vi "UHR-Fleezers Control (host) - 12.7b.vi"() -> ()   [LabVIEW 2012] (continued)
        n815 = case shown="True" w1258 {
          tunnel: w1261 -> [_ w1264]
          tunnel: "Fish for Tether" -> [_ w1263]
          frame False {
          }
          frame True {
            n816 = case shown="True" w1263 {
              selector: w1263 -> [w1267 w1273]
              tunnel: [w1267 w1273] -> w1262
              frame False {
              }
              frame True {
                n817 = local write "Scan axis 2"(TRUE) -> ()
                n818 = local write "Tether"(FALSE ("Tether")) -> ()
                n819 = local read "Flow ON during cal?"() -> (w1268:bool)
                n820 = property on="Trap Delta (MHz)" class="DigNum (strict)"("Val(Sgnl)"="Furthest Delta (MHz)") -> ()  [unwired: 2 in, 2 out]
                n821 = Or(x="Flow ON during \nfishing?", y=w1268) -> (x .or. y?=w1269:bool)
                n822 = Wait (ms)(milliseconds to wait=u32 500) -> ()  [unwired: 1 out]
                n823 = property on="Sample Channel\nFlow" class="Bool (strict)"("Val(Sgnl)"=w1269) -> ()  [unwired: 2 in, 2 out]
              }
            }
            n824 = node-c288() -> (w1266:T23)  [unwired: 1 in, 3 out]
            n825 = timed-loop "Oscillate AOD" {
              timing: w1266 -> [_]
              timing-out: [_] -> w1265
              tunnel: w1264 -> [w1283]
              tunnel: w1262 -> [w1276]
              i -> [w1285]
              stop <- w1282 stop-if-true
              n826 = node-c288() -> (w1284:i64)  [unwired: 1 out]
              n827 = flat-sequence {
                tunnel: w1285 -> [w1312]
                tunnel: w1284 -> [w1311]
                tunnel: w1283 -> [w1293]
                tunnel: w1276 -> [w1295]
                tunnel: [w1295] -> w1281
                tunnel: [w1294] -> w1280
                tunnel: [w1292] -> w1279
                tunnel: [w1289] -> w1277
                tunnel: w1281 -> [w1357]
                tunnel: w1280 -> [w1355]
                tunnel: w1279 -> [w1354]
                tunnel: [w1353] -> w1278
                tunnel: w1277 -> [w1352]
                tunnel: [w1429] -> w1282
                tunnel: w1278 -> [w1428]
                frame #0 {
                  # "w (rad/s)"
                  # "t (s)"
                  n828 = Divide(x=w1311, y=i64 1000) -> (x/y=w1286:dbl)
                  n829 = local read "BD 1 Frequency 2 (MHz)"() -> (w1288:dbl)
                  n830 = Multiply(x="Osc. freq. (Hz)", y=6.283185307179586) -> (x*y=w1309:dbl)
                  n831 = Multiply(x=w1286, y=w1312) -> (x*y=w1308:dbl)
                  n832 = Multiply(x=w1309, y=w1308) -> (x*y=w1291:dbl)
                  n833 = local read "BD 1 Frequency 1 (MHz)"() -> (w1297:dbl)
                  n834 = case shown="True" w1295 {
                    tunnel: w1291 -> [w1318 w1335]
                    tunnel: w1297 -> [_ w1343]
                    tunnel: w1288 -> [_ w1344]
                    tunnel: [w1315 w1339] -> w1287
                    tunnel: [FALSE w1320] -> w1292
                    tunnel: [0.0 w1331] -> w1289
                    frame False {
                      n835 = Sine(x=w1318) -> (sin(x)=w1316:dbl)
                      n836 = Multiply(x=w1316, y="Osc. amp. (MHz)") -> (x*y=w1315:dbl)
                    }
                    frame True {
                      # "trap position goes from 0 to 1 (0 is when it is furthest away, 1 is when closest)\nso we want to test for tether only when farther away, or x < 1"
                      # "quit if taking too long"
                      # "oscillate the trap"
                      # "Test for tether"
                      n837 = local read "Vec Mean of T1 T2"() -> (w1319:dbl[])
                      "Trigger Signal" <- w1319
                      n838 = Cosine(x=w1335) -> (cos(x)=w1347:dbl)
                      n839 = Subtract(x=w1344, y=w1343) -> (x-y=w1342:dbl)
                      n840 = Decrement(x=w1347) -> (x-1=w1346:dbl)
                      n841 = Subtract(x=w1342, y="Closest Delta (MHz)") -> (x-y=w1340:dbl)
                      n842 = Divide(x=w1346, y=-2.0) -> (x/y=w1330:dbl)
                      n843 = Greater?(x=w1319, y="Stop F (pN)") -> (0:w1337:bool[])
                      n844 = Multiply(x=w1330, y=w1340) -> (x*y=w1339:dbl)
                      n845 = Less?(x=w1330, y="Fish mask thresh") -> (x < y?=w1329:bool)
                      n846 = Boolean To (0,1)(Boolean=w1329) -> (0, 1=w1327:i16)
                      n847 = Multiply(x=w1327, y=w1319) -> (x*y=w1326:dbl[])
                      n848 = Divide(x=w1335, y=6.283185307179586) -> (x/y=w1334:dbl)
                      n849 = Round Toward +Infinity(x=w1334) -> (ceil(x): smallest int >= x=w1331:dbl)
                      "Attempts" <- w1331
                      n850 = Greater?(x=w1326, y="Stop F (pN) (mask)") -> (0:w1324:bool[])
                      n851 = Or Array Elements(Boolean array=w1337) -> (logical OR=w1322:bool)
                      n852 = Or Array Elements(Boolean array=w1324) -> (logical OR=w1321:bool)
                      n853 = Greater?(x=w1331, y="Attempt Limit") -> (0:w1333:bool)
                      n854 = case shown="True" w1333 {
                        frame False {
                        }
                        frame True {
                          n855 = local write "Fish for Tether"(FALSE ("Fish for Tether")) -> ()
                          n856 = call <vilib>:"Beep.vi"() -> ()  [unwired: 3 in, 9 out]
                          n857 = local read "Messages"() -> (w1349:string)
                          n858 = call "Update messages.vi"("Message to add"="Tether fishing timeout." ("Messages"), "Old message string"=w1349) -> ("New message string"=→"Messages":string)
                        }
                      }
                      n859 = Select(t=w1322, s="Normal (on) or masked test (off)", f=w1321) -> (s? t:f=w1320:bool)
                    }
                  }
                  n860 = local read "BD 2 Frequency 1 (MHz)"() -> (w1296:dbl)
                  n861 = Select(t=w1297, s="Scan axis 2", f=w1296) -> (s? t:f=w1300:dbl)
                  n862 = Add(x=w1287, y=w1300) -> (x+y=w1294:dbl)
                  n863 = Select(t=w1294, s="Scan axis 2", f=w1297) -> (s? t:f=w1303:dbl)
                  n864 = Select(t=w1296, s="Scan axis 2", f=w1294) -> (s? t:f=w1302:dbl)
                  n865 = local read "BD 2 Frequency 2 (MHz)"() -> (w1305:dbl)
                  n866 = local read "BD 2 Frequency 3 (MHz)"() -> (w1304:dbl)
                  n867 = local read "Y RF Frequency Limits (MHz)"() -> (w1298:T16)
                  n868 = local read "X RF Frequency Limits (MHz)"() -> (w1299:T16)
                  n869 = local read "BD 1 Frequency 3 (MHz)"() -> (w1306:dbl)
                  n870 = call "set RF board frequency - interlace.vi"("Board 2 Frequency Limits"=w1298, "Board 1 Frequency Limits"=w1299, "FPGA VI Reference In"=w1293, "Board 2 Frequency 3 (MHz)"=w1304, "Board 1 Frequency 3 (MHz)"=w1306, "Board 2 Frequency 2 (MHz)"=w1305, "Board 2 Frequency 1 (MHz)"=w1302, "Board 1 Frequency 2 (MHz)"=w1288, "Board 1 Frequency 1  (MHz)"=w1303) -> ()  [unwired: 1 in, 2 out]
                }
                frame #1 {
                  n871 = And(x=w1357, y=w1354) -> (x .and. y?=w1356:bool)
                  n872 = case "Only if were fishing and now formed tether" shown="True" w1356 {
                    tunnel: w1355 -> [w1359 w1374]
                    tunnel: [w1358 w1373] -> w1353
                    tunnel: w1352 -> [_ w1369]
                    frame False {
                      n873 = local read "Fish for Tether"() -> (w1358:bool)
                      n874 = case shown="False" w1358 {
                        tunnel: w1359 -> [w1360 _]
                        frame False {
                          n875 = property on="BD 1 Frequency 1 (MHz)" class="DigNum (strict)"("Val(Sgnl)"=w1360) -> ()  [unwired: 2 in, 2 out]
                        }
                        frame True {
                        }
                      }
                    }
                    frame True {
                      w1373 = FALSE ("Fish for Tether")
                      n876 = call <vilib>:"Beep.vi"() -> ()  [unwired: 3 in, 9 out]
                      n877 = Number To Decimal String(number=w1369, width (-)=i16 1) -> (decimal integer string=w1367:string)
                      n878 = Concatenate Strings("Formed tether in ", w1367, " attempt(s)." ("string")) -> (w1364:string)
                      n879 = local read "Messages"() -> (w1371:string)
                      n880 = local write "Fish for Tether"(w1373) -> ()
                      n881 = call "Update messages.vi"("Message to add"=w1364, "Old message string"=w1371) -> ("New message string"=w1370:string)
                      n882 = local write "Messages"(w1370) -> ()
                      n883 = Get Date/Time In Seconds() -> (seconds since 1Jan1904=→"Time tether formed":timestamp)
                      n884 = local read "Flow ON during cal?"() -> (w1361:bool)
                      n885 = property on="Sample Channel\nFlow" class="Bool (strict)"("Val(Sgnl)"=w1361) -> (error out=w1362:errorcluster)  [unwired: 2 in, 1 out]
                      n886 = case shown="\"2\", \"3\", \"4\", \"5\", \"6\"" "Then..." {
                        selector: "Then..." -> [_ w1377]
                        tunnel: w1374 -> [w1376 _]
                        tunnel: w1362 -> [_ _]
                        frame "1", Default {
                          n887 = property on="BD 1 Frequency 1 (MHz)" class="DigNum (strict)"("Val(Sgnl)"=w1376) -> ()  [unwired: 2 in, 2 out]
                        }
                        frame "2", "3", "4", "5", "6" {
                          n888 = flat-sequence {
                            tunnel: w1377 -> [w1379]
                            frame #0 {
                              n889 = property on="Trap Delta (MHz)" class="DigNum (strict)"("Val(Sgnl)"="Move to Delta 1 (MHz)") -> ()  [unwired: 2 in, 2 out]
                            }
                            frame #1 {
                              n890 = case shown="\"5\", \"6\"" w1379 {
                                selector: w1379 -> [w1382 w1392 _]
                                frame "3", "4" {
                                n891 = flat-sequence {
                                tunnel: w1382 -> [w1383]
                                tunnel: [w1383] -> w1380
                                tunnel: [w1385] -> w1381
                                tunnel: w1380 -> [w1385]
                                tunnel: w1381 -> [w1389]
                                frame #0 {
                                n892 = property on="Green Laser ON" class="Bool (strict)"("Val(Sgnl)"=TRUE ("Value (Signaling)")) -> ()  [unwired: 2 in, 2 out]
                                }
                                frame #1 {
                                n893 = Multiply(x="Wait Before Save (s)", y=u32 1000 ("x")) -> (x*y=w1387:u32)
                                n894 = Wait (ms)(milliseconds to wait=w1387) -> ()  [unwired: 1 out]
                                }
                                frame #2 {
                                n895 = property on="Start Saving" class="Bool (strict)"("Value"=TRUE ("Start Saving")) -> ()  [unwired: 2 in, 2 out]
                                n896 = case shown="\"4\"" w1389 {
                                frame Default {
                                }
                                frame "4" {
                                n897 = property on="Fl. Triggered..." class="Bool (strict)"("Val(Sgnl)"=TRUE ("Value (Signaling)")) -> ()  [unwired: 2 in, 2 out]
                                }
                                }
                                }
                                }
                                }
                                frame "5", "6" {
                                n898 = stacked-sequence {
                                tunnel: w1392 -> [_ _ _ _ _ _ w1404]
                                frame #0 {
                                n899 = Replace Array Subset(array=u32[] [0] ("Index Values"), new element="Raster Set Upon Tether", index=0) -> (w1393:u32[])
                                n900 = property on="Saved AOD Raster Scan Parameter Sets" class="Arr (strict)"("Index Values"=w1393) -> ()  [unwired: 2 in, 2 out]
                                }
                                frame #1 {
                                n901 = Wait (ms)(milliseconds to wait=u32 500) -> ()  [unwired: 1 out]
                                }
                                frame #2 {
                                n902 = property on="Load parameters" class="Bool (strict)"("Val(Sgnl)"=TRUE ("Value (Signaling)")) -> ()  [unwired: 2 in, 2 out]
                                n903 = case shown="True" "Green ON During Raster" {
                                frame False {
                                }
                                frame True {
                                n904 = property on="Green Laser ON" class="Bool (strict)"("Val(Sgnl)"=TRUE ("Value (Signaling)")) -> ()  [unwired: 2 in, 2 out]
                                }
                                }
                                }
                                frame #3 {
                                n905 = Wait (ms)(milliseconds to wait=u32 500) -> ()  [unwired: 1 out]
                                }
                                frame #4 {
                                n906 = property on="Trap Raster Scan" class="Bool (strict)"("Val(Sgnl)"=TRUE ("Value (Signaling)")) -> ()  [unwired: 2 in, 2 out]
                                }
                                frame #5 {
                                n907 = Wait (ms)(milliseconds to wait=u32 2000) -> ()  [unwired: 1 out]
                                }
                                frame #6 {
                                n908 = flat-sequence {
                                tunnel: w1404 -> [w1411]
                                frame #0 {
                                n909 = while {
                                stop <- w1407 stop-if-true
                                n910 = local read "Raster Scanning..."() -> (w1406:bool)
                                n911 = local read "Saving..."() -> (w1409:bool)
                                n912 = Wait (ms)(milliseconds to wait=u32 100) -> ()  [unwired: 1 out]
                                n913 = Not(x=w1409) -> (.not. x?=w1408:bool)
                                n914 = Not(x=w1406) -> (.not. x?=w1405:bool)
                                n915 = And(x=w1408, y=w1405) -> (x .and. y?=w1407:bool)
                                }
                                }
                                frame #1 {
                                n916 = local read "Tether"() -> (w1412:bool)
                                n917 = case shown="True" w1412 {
                                tunnel: w1411 -> [_ w1414]
                                frame False {
                                n918 = property on="Fish for Tether" class="Bool (strict)"("Val(Sgnl)"="Fish again after \nraster break?") -> ()  [unwired: 2 in, 2 out]
                                }
                                frame True {
                                n919 = stacked-sequence {
                                tunnel: w1414 -> [_ w1418 _ _]
                                frame #0 {
                                n920 = property on="Trap Delta (MHz)" class="DigNum (strict)"("Val(Sgnl)"="Move to Delta 2 (MHz)") -> ()  [unwired: 2 in, 2 out]
                                n921 = case shown="True" "Flow ON after\ntether testing?" {
                                frame False {
                                }
                                frame True {
                                n922 = property on="Sample Channel\nFlow" class="Bool (strict)"("Val(Sgnl)"=TRUE ("Value (Signaling)")) -> ()  [unwired: 2 in, 2 out]
                                }
                                }
                                }
                                frame #1 {
                                n923 = flat-sequence {
                                tunnel: w1418 -> [w1420]
                                frame #0 {
                                n924 = Wait (ms)(milliseconds to wait=u32 500) -> ()  [unwired: 1 out]
                                }
                                frame #1 {
                                n925 = case shown="\"6\"" w1420 {
                                frame Default {
                                }
                                frame "6" {
                                n926 = property on="Green Laser ON" class="Bool (strict)"("Val(Sgnl)"=TRUE ("Green Laser ON/Interlacing")) -> ()  [unwired: 2 in, 2 out]
                                }
                                }
                                }
                                frame #2 {
                                n927 = Wait (ms)(milliseconds to wait=u32 500) -> ()  [unwired: 1 out]
                                }
                                frame #3 {
                                n928 = local write "Start Saving"("Save at end (5, 6)") -> ()
                                }
                                }
                                }
                                frame #2 {
                                n929 = local read "Bead Sep. Int. Time (s)"() -> (w1426:dbl)
                                n930 = Multiply(x=w1426, y=1000.0) -> (x*y=w1425:dbl)
                                n931 = Wait (ms)(milliseconds to wait=w1425) -> ()  [unwired: 1 out]
                                }
                                frame #3 {
                                n932 = property on="Remove Offset" class="Bool (strict)"("Val(Sgnl)"=TRUE ("Value (Signaling)")) -> ()  [unwired: 2 in, 2 out]
                                }
                                }
                                }
                                }
                                }
                                }
                                }
                                }
                                }
                                frame "2", Default {
                                }
                              }
                            }
                          }
                        }
                      }
                      "Tether" <- "Tether Alarm?"
                    }
                  }
                }
                frame #2 {
                  n933 = local read "Oscillate Set 1"() -> (w1433:bool)
                  n934 = local read "Stop All"() -> (w1431:bool)
                  n935 = Or(x=w1433, y=w1428) -> (x .or. y?=w1430:bool)
                  n936 = Not(x=w1430) -> (.not. x?=w1432:bool)
                  n937 = Compound Arithmetic op=OR(w1431, w1432) -> (w1429:bool)
                }
              }
              n938 = node-c288() -> ()  [unwired: 2 out]
            }
            n939 = node-c288(w1265) -> ()  [unwired: 1 out]
          }
        }
      }
      event "Fl. Triggered...": Value Change {
        n940 = event-data() -> ()  [unwired: 7 out]
        n941 = case shown="True" "Fl. Triggered..." {
          frame False {
          }
          frame True {
            n942 = node-c288() -> (w1444:T23)  [unwired: 4 out]
            n943 = timed-loop {
              timing: w1444 -> [_]
              timing-out: [_] -> w1443
              tunnel: "Action" -> [w1452]
              shift-right: [w1449] -> _
              shift-left: u8 255 -> [w1451]
              shift-right: [w1446] -> _
              shift-left: 255 -> [w1448]
              stop <- w1445 stop-if-true
              # "Reset confocal spot"
              n944 = node-c288() -> ()  [unwired: 2 out]
              n945 = flat-sequence {
                tunnel: w1452 -> [w1472]
                tunnel: w1451 -> [w1471]
                tunnel: [w1470] -> w1450
                tunnel: w1448 -> [w1457]
                tunnel: [w1456] -> w1447
                tunnel: [w1851] -> w1445
                tunnel: w1450 -> [w1850]
                tunnel: [w1850] -> w1449
                tunnel: [w1849] -> w1446
                tunnel: w1447 -> [w1849]
                frame #0 {
                  n946 = local read "Delta Fl. 2"() -> (w1469:dbl)
                  n947 = local read "Delta Fl. 1"() -> (w1464:dbl)
                  n948 = Multiply(x="Fl. Delta Thresh. (kHz)", y=1000.0) -> (x*y=w1459:dbl)
                  n949 = Select(t=w1464, s="APD to Watch", f=w1469) -> (s? t:f=w1460:dbl)
                  n950 = Greater?(x=w1460, y=w1459) -> (0:w1465:bool)
                  n951 = Or(x="Force Yank", y=w1465) -> (x .or. y?=w1463:bool)
                  n952 = And(x=w1463, y="Yank when?") -> (x .and. y?=w1461:bool)
                  n953 = case shown="False" w1461 {
                    tunnel: w1472 -> [w1475 w1676]
                    tunnel: w1471 -> [w1477 w1672]
                    tunnel: [w1477 w1670] -> w1470
                    tunnel: w1460 -> [w1483 _]
                    tunnel: w1459 -> [w1482 _]
                    tunnel: "Force Yank" -> [w1480 _]
                    tunnel: w1457 -> [w1479 w1669]
                    tunnel: [w1478 w1669] -> w1456
                    frame False {
                      n954 = Negate(x=w1482) -> (-x=w1474:dbl)
                      n955 = local write "Fl. High"(TRUE ("Fl. High")) -> ()
                      n956 = Less?(x=w1483, y=w1474) -> (x < y?=w1481:bool)
                      n957 = Or(x=w1480, y=w1481) -> (x .or. y?=w1476:bool)
                      n958 = case shown="True" w1476 {
                        tunnel: w1479 -> [w1484 w1494]
                        tunnel: [w1484 w1493] -> w1478
                        tunnel: w1475 -> [_ w1492]
                        frame False {
                        }
                        frame True {
                          n959 = flat-sequence {
                            tunnel: w1494 -> [w1500]
                            tunnel: w1492 -> [w1497]
                            tunnel: [w1499] -> w1491
                            tunnel: [w1498] -> w1490
                            tunnel: [w1497] -> w1489
                            tunnel: w1488 -> [w1496]
                            tunnel: [w1496] -> w1487
                            tunnel: w1486 -> [w1495]
                            tunnel: [w1495] -> w1485
                            tunnel: [w1571] -> w1493
                            tunnel: w1491 -> [w1571]
                            tunnel: w1490 -> [w1570]
                            tunnel: w1489 -> [w1569]
                            tunnel: w1487 -> [w1568]
                            tunnel: w1485 -> [w1567]
                            frame #0 {
                              n960 = call <vilib>:"Beep.vi"() -> ()  [unwired: 12 in]
                              n961 = local write "Waiting"(FALSE ("Waiting")) -> ()
                              n962 = Increment(x=w1500) -> (x+1=w1499:i32)
                              n963 = case shown="\"Image\"" w1497 {
                                tunnel: w1499 -> [_ w1505 _]
                                frame "Alarm", Default {
                                }
                                frame "Yank" {
                                n964 = flat-sequence {
                                tunnel: w1505 -> [w1508]
                                tunnel: [w1507] -> w1504
                                tunnel: [w1506] -> w1503
                                tunnel: w1504 -> [w1518]
                                tunnel: w1503 -> [w1519]
                                frame #0 {
                                n965 = local read "Yank Delay (s)"() -> (w1511:dbl)
                                n966 = local read "N Array El"() -> (w1506:u8)
                                n967 = Quotient & Remainder(x=w1508, y=w1506) -> (x-y*floor(x/y)=w1507:i32)  [unwired: 1 out]
                                n968 = Multiply(x=w1511, y=1000.0) -> (x*y=w1509:dbl)
                                n969 = Wait (ms)(milliseconds to wait=w1509) -> ()  [unwired: 1 out]
                                }
                                frame #1 {
                                n970 = local read "Yank to which?"() -> (w1513:bool)
                                n971 = local read "Random Choice"() -> (w1523:bool)
                                n972 = local read "Yank to Trap Delta (MHz)"() -> (w1516:dbl[])
                                n973 = local read "Yank to SP"() -> (w1517:dbl[])
                                n974 = Random Number (0-1)() -> (number: 0 to 1=w1522:dbl)
                                n975 = Multiply(x=w1519, y=w1522) -> (x*y=w1521:dbl)
                                n976 = Round Toward -Infinity(1:w1521) -> (0:w1520:dbl)
                                n977 = Select(t=w1520, s=w1523, f=w1518) -> (s? t:f=w1514:dbl)
                                n978 = Select(t=w1516, s=w1513, f=w1517) -> (s? t:f=w1515:dbl[])
                                n979 = Index Array(array=w1515, index=w1514) -> (element=w1512:dbl)
                                n980 = case shown="True" w1513 {
                                tunnel: w1512 -> [w1524 w1551]
                                frame False {
                                n981 = flat-sequence {
                                tunnel: w1524 -> [w1525]
                                frame #0 {
                                n982 = property on="Trap Pos FB SP" class="DigNum (strict)"("Val(Sgnl)"=w1525) -> ()  [unwired: 2 in, 2 out]
                                }
                                frame #1 {
                                n983 = Wait (ms)(milliseconds to wait=u32 700) -> ()  [unwired: 1 out]
                                }
                                frame #2 {
                                n984 = local read "Action (%)"() -> (w1530:dbl)
                                n985 = Absolute Value(x=w1530) -> (abs(x)=w1529:dbl)
                                n986 = Greater?(x=w1529, y=70.0) -> (0:w1527:bool)
                                n987 = property on="Remove Action Offset" class="Bool (strict)"("Val(Sgnl)"=w1527) -> ()  [unwired: 2 in, 2 out]
                                }
                                frame #3 {
                                n988 = for {
                                N: 4 -> [_]
                                n989 = flat-sequence {
                                frame #0 {
                                n990 = Wait (ms)(milliseconds to wait=u32 500) -> ()  [unwired: 1 out]
                                }
                                frame #1 {
                                n991 = local read "Action (%)"() -> (w1536:dbl)
                                n992 = Absolute Value(x=w1536) -> (abs(x)=w1535:dbl)
                                n993 = Greater?(x=w1535, y=70.0) -> (0:w1533:bool)
                                n994 = property on="Remove Action Offset" class="Bool (strict)"("Val(Sgnl)"=w1533) -> ()  [unwired: 2 in, 2 out]
                                }
                                }
                                }
                                }
                                frame #4 {
                                n995 = Wait (ms)(milliseconds to wait=u32 500) -> ()  [unwired: 1 out]
                                }
                                frame #5 {
                                n996 = local read "Mean"() -> (w1544:dbl)
                                n997 = Greater?(x=w1544, y=11.0) -> (0:w1538:bool)
                                n998 = Not(x=w1538) -> (.not. x?=w1539:bool)
                                n999 = And(x=w1539, y="Shift confocal") -> (x .and. y?=w1541:bool)
                                n1000 = And(x=w1538, y="Shift confocal") -> (x .and. y?=w1542:bool)
                                n1001 = case shown="True" w1542 {
                                frame False {
                                }
                                frame True {
                                n1002 = local read "Confocal Y 2 (V)"() -> (w1548:dbl)
                                n1003 = local read "Confocal X 2 (V)"() -> (w1547:dbl)
                                n1004 = property on="AO1" class="Slide (strict)"("Val(Sgnl)"=w1548) -> ()  [unwired: 2 in, 2 out]
                                n1005 = property on="AO2" class="Slide (strict)"("Val(Sgnl)"=w1547) -> ()  [unwired: 2 in, 2 out]
                                }
                                }
                                n1006 = case shown="True" w1541 {
                                frame False {
                                }
                                frame True {
                                n1007 = local read "Confocal Y 1 (V)"() -> (w1546:dbl)
                                n1008 = local read "Confocal X 1 (V)"() -> (w1545:dbl)
                                n1009 = property on="AO1" class="Slide (strict)"("Val(Sgnl)"=w1546) -> ()  [unwired: 2 in, 2 out]
                                n1010 = property on="AO2" class="Slide (strict)"("Val(Sgnl)"=w1545) -> ()  [unwired: 2 in, 2 out]
                                }
                                }
                                }
                                frame #6 {
                                n1011 = Wait (ms)(milliseconds to wait=u32 1500) -> ()  [unwired: 1 out]
                                }
                                frame #7 {
                                n1012 = property on="Rem fb disp offset" class="Bool (strict)"("Val(Sgnl)"=TRUE ("Value (Signaling)")) -> ()  [unwired: 2 in, 2 out]
                                }
                                }
                                }
                                frame True {
                                n1013 = flat-sequence {
                                tunnel: w1551 -> [w1552]
                                frame #0 {
                                n1014 = property on="Trap Delta (MHz)" class="DigNum (strict)"("Val(Sgnl)"=w1552) -> ()  [unwired: 2 in, 2 out]
                                }
                                frame #1 {
                                n1015 = Wait (ms)(milliseconds to wait=u32 500) -> ()  [unwired: 1 out]
                                }
                                frame #2 {
                                n1016 = local read "Shift confocal"() -> (w1558:bool)
                                n1017 = local read "Mean"() -> (w1560:dbl)
                                n1018 = Greater?(x=w1560, y=11.0) -> (0:w1557:bool)
                                n1019 = Not(x=w1557) -> (.not. x?=w1556:bool)
                                n1020 = And(x=w1556, y=w1558) -> (x .and. y?=w1554:bool)
                                n1021 = And(x=w1557, y=w1558) -> (x .and. y?=w1555:bool)
                                n1022 = case shown="True" w1555 {
                                frame False {
                                }
                                frame True {
                                n1023 = local read "Confocal Y 2 (V)"() -> (w1564:dbl)
                                n1024 = local read "Confocal X 2 (V)"() -> (w1563:dbl)
                                n1025 = property on="AO2" class="Slide (strict)"("Val(Sgnl)"=w1563) -> ()  [unwired: 2 in, 2 out]
                                n1026 = property on="AO1" class="Slide (strict)"("Val(Sgnl)"=w1564) -> ()  [unwired: 2 in, 2 out]
                                }
                                }
                                n1027 = case shown="True" w1554 {
                                frame False {
                                }
                                frame True {
                                n1028 = local read "Confocal X 1 (V)"() -> (w1561:dbl)
                                n1029 = local read "Confocal Y 1 (V)"() -> (w1562:dbl)
                                n1030 = property on="AO2" class="Slide (strict)"("Val(Sgnl)"=w1561) -> ()  [unwired: 2 in, 2 out]
                                n1031 = property on="AO1" class="Slide (strict)"("Val(Sgnl)"=w1562) -> ()  [unwired: 2 in, 2 out]
                                }
                                }
                                }
                                }
                                }
                                }
                                }
                                }
                                }
                                frame "Image" {
                                n1032 = property on="Confocal Image" class="Bool (strict)"("Val(Sgnl)"=TRUE ("Value (Signaling)")) -> ()  [unwired: 2 in, 2 out]
                                }
                              }
                              n1033 = local write "Fl. High"(FALSE ("Fl. High")) -> ()
                              n1034 = local read "Time (s)"() -> (w1498:dbl)
                            }
                            frame #1 {
                              n1035 = case shown="True" "Auto F Reset" {
                                tunnel: w1570 -> [_ w1575]
                                tunnel: w1569 -> [_ w1574]
                                tunnel: w1568 -> [_ w1573]
                                tunnel: w1567 -> [_ w1572]
                                frame False {
                                }
                                frame True {
                                n1036 = node-c288() -> (w1577:T23)  [unwired: 4 in]
                                n1037 = timed-loop {
                                timing: w1577 -> [_]
                                timing-out: [_] -> w1576
                                tunnel: w1575 -> [w1582]
                                tunnel: w1574 -> [w1581]
                                tunnel: w1573 -> [w1580]
                                tunnel: w1572 -> [w1579]
                                stop <- w1578 stop-if-true
                                n1038 = node-c288() -> ()  [unwired: 1 in, 1 out]
                                n1039 = local read "Fl. Delta Thresh. (kHz)"() -> (w1591:dbl)
                                n1040 = local read "APD to Watch"() -> (w1592:bool)
                                n1041 = local read "Delta Fl. 1"() -> (w1593:dbl)
                                n1042 = local read "Delta Fl. 2"() -> (w1594:dbl)
                                n1043 = local read "Fl. Triggered..."() -> (w1585:bool)
                                n1044 = local read "Stop All"() -> (w1586:bool)
                                n1045 = local read "Reset Force"() -> (w1584:bool)
                                n1046 = Multiply(x=w1591, y=1000.0) -> (x*y=w1589:dbl)
                                n1047 = Select(t=w1593, s=w1592, f=w1594) -> (s? t:f=w1588:dbl)
                                n1048 = Not(x=w1585) -> (.not. x?=w1583:bool)
                                n1049 = Greater?(x=w1588, y=w1589) -> (0:w1587:bool)
                                n1050 = Compound Arithmetic op=OR(w1587, w1586, w1583, w1584) -> (w1578:bool)
                                n1051 = case shown="True" w1578 {
                                tunnel: w1582 -> [_ w1598]
                                tunnel: w1581 -> [_ w1602]
                                tunnel: w1580 -> [_ w1601]
                                tunnel: w1579 -> [_ w1600]
                                frame False {
                                }
                                frame True {
                                n1052 = case shown="\"Yank\"" w1602 {
                                tunnel: w1601 -> [_ w1612]
                                tunnel: w1600 -> [_ w1610]
                                frame "Image", Default {
                                }
                                frame "Yank" {
                                n1053 = flat-sequence {
                                tunnel: [w1615] -> w1613
                                tunnel: w1612 -> [w1615]
                                tunnel: [w1614] -> w1611
                                tunnel: w1610 -> [w1614]
                                tunnel: w1613 -> [w1621]
                                tunnel: w1611 -> [w1619]
                                frame #0 {
                                n1054 = local read "Yank Delay (s)"() -> (w1618:dbl)
                                n1055 = Multiply(x=w1618, y=1000.0) -> (x*y=w1616:dbl)
                                n1056 = Wait (ms)(milliseconds to wait=w1616) -> ()  [unwired: 1 out]
                                }
                                frame #1 {
                                n1057 = local read "Yank to which?"() -> (w1620:bool)
                                n1058 = case shown="False" w1620 {
                                tunnel: w1621 -> [_ w1649]
                                tunnel: w1619 -> [w1622 _]
                                frame False {
                                n1059 = flat-sequence {
                                tunnel: w1622 -> [w1623]
                                frame #0 {
                                n1060 = property on="Trap Pos FB SP" class="DigNum (strict)"("Val(Sgnl)"=w1623) -> ()  [unwired: 2 in, 2 out]
                                }
                                frame #1 {
                                n1061 = Wait (ms)(milliseconds to wait=u32 700) -> ()  [unwired: 1 out]
                                }
                                frame #2 {
                                n1062 = local read "Action (%)"() -> (w1628:dbl)
                                n1063 = Absolute Value(x=w1628) -> (abs(x)=w1627:dbl)
                                n1064 = Greater?(x=w1627, y=70.0) -> (0:w1625:bool)
                                n1065 = property on="Remove Action Offset" class="Bool (strict)"("Val(Sgnl)"=w1625) -> ()  [unwired: 2 in, 2 out]
                                }
                                frame #3 {
                                n1066 = for {
                                N: 4 -> [_]
                                n1067 = flat-sequence {
                                frame #0 {
                                n1068 = Wait (ms)(milliseconds to wait=u32 500) -> ()  [unwired: 1 out]
                                }
                                frame #1 {
                                n1069 = local read "Action (%)"() -> (w1634:dbl)
                                n1070 = Absolute Value(x=w1634) -> (abs(x)=w1633:dbl)
                                n1071 = Greater?(x=w1633, y=70.0) -> (0:w1631:bool)
                                n1072 = property on="Remove Action Offset" class="Bool (strict)"("Val(Sgnl)"=w1631) -> ()  [unwired: 2 in, 2 out]
                                }
                                }
                                }
                                }
                                frame #4 {
                                n1073 = Wait (ms)(milliseconds to wait=u32 500) -> ()  [unwired: 1 out]
                                }
                                frame #5 {
                                n1074 = local read "Shift confocal"() -> (w1639:bool)
                                n1075 = local read "Mean"() -> (w1642:dbl)
                                n1076 = Greater?(x=w1642, y=11.0) -> (0:w1638:bool)
                                n1077 = Not(x=w1638) -> (.not. x?=w1637:bool)
                                n1078 = And(x=w1638, y=w1639) -> (x .and. y?=w1640:bool)
                                n1079 = And(x=w1637, y=w1639) -> (x .and. y?=w1636:bool)
                                n1080 = case shown="True" w1640 {
                                frame False {
                                }
                                frame True {
                                n1081 = local read "Confocal X 2 (V)"() -> (w1645:dbl)
                                n1082 = local read "Confocal Y 2 (V)"() -> (w1646:dbl)
                                n1083 = property on="AO2" class="Slide (strict)"("Val(Sgnl)"=w1645) -> ()  [unwired: 2 in, 2 out]
                                n1084 = property on="AO1" class="Slide (strict)"("Val(Sgnl)"=w1646) -> ()  [unwired: 2 in, 2 out]
                                }
                                }
                                n1085 = case shown="True" w1636 {
                                frame False {
                                }
                                frame True {
                                n1086 = local read "Confocal Y 1 (V)"() -> (w1644:dbl)
                                n1087 = local read "Confocal X 1 (V)"() -> (w1643:dbl)
                                n1088 = property on="AO1" class="Slide (strict)"("Val(Sgnl)"=w1644) -> ()  [unwired: 2 in, 2 out]
                                n1089 = property on="AO2" class="Slide (strict)"("Val(Sgnl)"=w1643) -> ()  [unwired: 2 in, 2 out]
                                }
                                }
                                }
                                frame #6 {
                                n1090 = Wait (ms)(milliseconds to wait=u32 1500) -> ()  [unwired: 1 out]
                                }
                                frame #7 {
                                n1091 = property on="Rem fb disp offset" class="Bool (strict)"("Val(Sgnl)"=TRUE ("Value (Signaling)")) -> ()  [unwired: 2 in, 2 out]
                                }
                                }
                                }
                                frame True {
                                n1092 = flat-sequence {
                                tunnel: w1649 -> [w1650]
                                frame #0 {
                                n1093 = property on="Trap Delta (MHz)" class="DigNum (strict)"("Val(Sgnl)"=w1650) -> ()  [unwired: 2 in, 2 out]
                                }
                                frame #1 {
                                n1094 = Wait (ms)(milliseconds to wait=u32 500) -> ()  [unwired: 1 out]
                                }
                                frame #2 {
                                n1095 = local read "Shift confocal"() -> (w1656:bool)
                                n1096 = local read "Mean"() -> (w1657:dbl)
                                n1097 = Greater?(x=w1657, y=11.0) -> (0:w1655:bool)
                                n1098 = And(x=w1655, y=w1656) -> (x .and. y?=w1653:bool)
                                n1099 = Not(x=w1655) -> (.not. x?=w1654:bool)
                                n1100 = And(x=w1654, y=w1656) -> (x .and. y?=w1652:bool)
                                n1101 = case shown="True" w1653 {
                                frame False {
                                }
                                frame True {
                                n1102 = local read "Confocal Y 2 (V)"() -> (w1662:dbl)
                                n1103 = local read "Confocal X 2 (V)"() -> (w1661:dbl)
                                n1104 = property on="AO1" class="Slide (strict)"("Val(Sgnl)"=w1662) -> ()  [unwired: 2 in, 2 out]
                                n1105 = property on="AO2" class="Slide (strict)"("Val(Sgnl)"=w1661) -> ()  [unwired: 2 in, 2 out]
                                }
                                }
                                n1106 = case shown="True" w1652 {
                                frame False {
                                }
                                frame True {
                                n1107 = local read "Confocal Y 1 (V)"() -> (w1660:dbl)
                                n1108 = local read "Confocal X 1 (V)"() -> (w1659:dbl)
                                n1109 = property on="AO2" class="Slide (strict)"("Val(Sgnl)"=w1659) -> ()  [unwired: 2 in, 2 out]
                                n1110 = property on="AO1" class="Slide (strict)"("Val(Sgnl)"=w1660) -> ()  [unwired: 2 in, 2 out]
                                }
                                }
                                }
                                }
                                }
                                }
                                }
                                }
                                }
                                }
                                n1111 = local read "Time (s)"() -> (w1597:dbl)
                                n1112 = Subtract(x=w1598, y=w1597) -> (x-y=w1609:dbl)
                                n1113 = Number To Decimal String(number=w1609, width (-)=i16 0) -> (decimal integer string=w1607:string)
                                n1114 = Concatenate Strings(w1607, " s fluorescence event") -> (w1604:string)
                                n1115 = local read "Messages"() -> (w1605:string)
                                n1116 = local write "Duration (s)"(w1609) -> ()
                                n1117 = call "Update messages.vi"("Message to add"=w1604, "Old message string"=w1605) -> ("New message string"=w1603:string)
                                n1118 = local write "Messages"(w1603) -> ()
                                n1119 = call <vilib>:"Beep.vi"() -> ()  [unwired: 12 in]
                                n1120 = local write "Reset Force"(FALSE ("Force Reset")) -> ()
                                n1121 = local write "Fl. High"(TRUE ("Fl. High")) -> ()
                                n1122 = local write "Waiting"(TRUE ("Waiting")) -> ()
                                }
                                }
                                n1123 = node-c288() -> ()  [unwired: 1 in, 1 out]
                                }
                                n1124 = node-c288(w1576) -> ()  [unwired: 1 out]
                                }
                              }
                            }
                          }
                          n1125 = local read "Trap Delta (MHz)"() -> (w1488:dbl)
                          n1126 = local read "Trap Pos FB SP"() -> (w1486:fxp<+/-,16,1>)
                        }
                      }
                    }
                    frame True {
                      n1127 = flat-sequence {
                        tunnel: w1673 -> [w1683]
                        tunnel: [w1683] -> w1677
                        tunnel: w1676 -> [w1682]
                        tunnel: [w1682] -> w1675
                        tunnel: [w1681] -> w1674
                        tunnel: w1672 -> [w1680]
                        tunnel: [w1679] -> w1671
                        tunnel: w1668 -> [w1678]
                        tunnel: [w1678] -> w1667
                        tunnel: w1677 -> [w1753]
                        tunnel: w1675 -> [w1752]
                        tunnel: w1674 -> [w1751]
                        tunnel: w1671 -> [w1750]
                        tunnel: w1667 -> [w1749]
                        tunnel: [w1750] -> w1670
                        frame #0 {
                          n1128 = call <vilib>:"Beep.vi"() -> ()  [unwired: 3 in, 9 out]
                          n1129 = local write "Waiting"(FALSE ("Waiting")) -> ()
                          n1130 = Increment(x=w1680) -> (x+1=w1679:u8)
                          n1131 = case shown="\"Yank\"" w1682 {
                            tunnel: w1679 -> [_ _ w1689]
                            frame "Image" {
                              n1132 = property on="Confocal Image" class="Bool (strict)"("Val(Sgnl)"=TRUE ("Value (Signaling)")) -> ()  [unwired: 2 in, 2 out]
                            }
                            frame "Alarm", Default {
                            }
                            frame "Yank" {
                              n1133 = flat-sequence {
                                tunnel: w1689 -> [w1692]
                                tunnel: [w1691] -> w1688
                                tunnel: ["N Array El"] -> w1687
                                tunnel: w1688 -> [w1706]
                                tunnel: w1687 -> [w1702]
                                frame #0 {
                                n1134 = Multiply(x="Yank Delay (s)", y=1000.0) -> (x*y=w1695:dbl)
                                n1135 = Quotient & Remainder(x=w1692, y="N Array El") -> (x-y*floor(x/y)=w1691:u8)  [unwired: 1 out]
                                n1136 = Wait (ms)(milliseconds to wait=w1695) -> ()  [unwired: 1 out]
                                }
                                frame #1 {
                                n1137 = Random Number (0-1)() -> (number: 0 to 1=w1703:dbl)
                                n1138 = Multiply(x=w1702, y=w1703) -> (x*y=w1701:dbl)
                                n1139 = Round Toward -Infinity(1:w1701) -> (0:w1700:dbl)
                                n1140 = Select(t=w1700, s="Random Choice", f=w1706) -> (s? t:f=w1704:dbl)
                                n1141 = Select(t="Yank to Trap Delta (MHz)", s="Yank to which?", f="Yank to SP") -> (s? t:f=w1697:dbl[])
                                n1142 = Index Array(array=w1697, index=w1704) -> (element=w1707:dbl)
                                n1143 = case shown="False" "Yank to which?" {
                                tunnel: w1707 -> [w1708 w1734]
                                frame False {
                                n1144 = flat-sequence {
                                tunnel: w1708 -> [w1709]
                                frame #0 {
                                n1145 = property on="Trap Pos FB SP" class="DigNum (strict)"("Val(Sgnl)"=w1709) -> ()  [unwired: 2 in, 2 out]
                                }
                                frame #1 {
                                n1146 = Wait (ms)(milliseconds to wait=u32 700) -> ()  [unwired: 1 out]
                                }
                                frame #2 {
                                n1147 = local read "Action (%)"() -> (w1714:dbl)
                                n1148 = Absolute Value(x=w1714) -> (abs(x)=w1713:dbl)
                                n1149 = Greater?(x=w1713, y=70.0) -> (0:w1711:bool)
                                n1150 = property on="Remove Action Offset" class="Bool (strict)"("Val(Sgnl)"=w1711) -> ()  [unwired: 2 in, 2 out]
                                }
                                frame #3 {
                                n1151 = for {
                                N: 4 -> [_]
                                n1152 = flat-sequence {
                                frame #0 {
                                n1153 = Wait (ms)(milliseconds to wait=u32 500) -> ()  [unwired: 1 out]
                                }
                                frame #1 {
                                n1154 = local read "Action (%)"() -> (w1720:dbl)
                                n1155 = Absolute Value(x=w1720) -> (abs(x)=w1719:dbl)
                                n1156 = Greater?(x=w1719, y=70.0) -> (0:w1717:bool)
                                n1157 = property on="Remove Action Offset" class="Bool (strict)"("Val(Sgnl)"=w1717) -> ()  [unwired: 2 in, 2 out]
                                }
                                }
                                }
                                }
                                frame #4 {
                                n1158 = local read "Shift confocal"() -> (w1724:bool)
                                n1159 = local read "Mean"() -> (w1727:dbl)
                                n1160 = Greater?(x=w1727, y=11.0) -> (0:w1723:bool)
                                n1161 = Not(x=w1723) -> (.not. x?=w1722:bool)
                                n1162 = And(x=w1722, y=w1724) -> (x .and. y?=w1721:bool)
                                n1163 = And(x=w1723, y=w1724) -> (x .and. y?=w1725:bool)
                                n1164 = case shown="True" w1725 {
                                frame False {
                                }
                                frame True {
                                n1165 = local read "Confocal X 2 (V)"() -> (w1730:dbl)
                                n1166 = local read "Confocal Y 2 (V)"() -> (w1731:dbl)
                                n1167 = property on="AO2" class="Slide (strict)"("Val(Sgnl)"=w1730) -> ()  [unwired: 2 in, 2 out]
                                n1168 = property on="AO1" class="Slide (strict)"("Val(Sgnl)"=w1731) -> ()  [unwired: 2 in, 2 out]
                                }
                                }
                                n1169 = case shown="True" w1721 {
                                frame False {
                                }
                                frame True {
                                n1170 = local read "Confocal X 1 (V)"() -> (w1728:dbl)
                                n1171 = local read "Confocal Y 1 (V)"() -> (w1729:dbl)
                                n1172 = property on="AO1" class="Slide (strict)"("Val(Sgnl)"=w1729) -> ()  [unwired: 2 in, 2 out]
                                n1173 = property on="AO2" class="Slide (strict)"("Val(Sgnl)"=w1728) -> ()  [unwired: 2 in, 2 out]
                                }
                                }
                                }
                                frame #5 {
                                n1174 = Wait (ms)(milliseconds to wait=u32 1500) -> ()  [unwired: 1 out]
                                }
                                frame #6 {
                                n1175 = property on="Rem fb disp offset" class="Bool (strict)"("Val(Sgnl)"=TRUE ("Value (Signaling)")) -> ()  [unwired: 2 in, 2 out]
                                }
                                }
                                }
                                frame True {
                                n1176 = flat-sequence {
                                tunnel: w1734 -> [w1735]